vi "Joystick and Camera SHIH VPC- external Connection.vi"(0 "Motion in":refnum<class "Motion.lvclass">, 1 "XYZTheta":dbl[](array[numeric]), 2 "Measurement Point":string, 3 "Inital GO":bool=TRUE) -> (7 "Motion out":refnum<class "Motion.lvclass">, 8 "Sum":dbl[](array[numeric]), 9 "Gantry":dbl[](array[numeric]), 10 "error out":errorcluster)   [LabVIEW 2016]
uses:
  Classes/Controllers/Motion/Copy of Motion Folder/Motion.lvclass
  Classes/Controllers/Camera/Copy of Camera Folder/Machine Vision.ctl
  Classes/Controllers/Camera/Copy of Camera Folder/Camera.lvclass
  Classes/Controllers/Camera/Copy of Controller Folder/Controller.lvclass
panel:
  in  "case NN":dbl=0.001 format="%#_13g"
  in  "case NY":dbl=0.003 format="%#_13g"
  in  "?":bool
  in  "operation go":dbl[](array[numeric]) format="%#_9g"
  in  "case YN":dbl=0.01 format="%#_13g"
  in  "case YY":dbl=0.1 format="%#_13g"
  in  "?":bool=TRUE
  in  "step":dbl=15.0
  in  "Z go up":bool
  in  "Z go down":bool
  in  "Machine Vision":T1
  in  "object goes left":bool
  in  "object goes right":bool
  in  "object goes down":bool
  in  "object goes up":bool
  in  "Z go up 25 um":bool
  in  "Z go down 25 um":bool
  in  "Z go up 0.05 mm":bool
  in  "Z go down 0.05 mm":bool
  in  "Z go  up 0.1 mm":bool
  in  "Z go down 0.1 mm":bool
  in  "Machine Vision 2":T1=enum."None"
  out "Image 2":T2(plugin-control)
  out "Focus Index":dbl[](array[numeric])
  in  "interval":dbl=0.005
  out "Score":dbl[](array[numeric])
  out "Waveform Graph":dbl[](graph)
  in  "focus":bool
  out "Numeric":dbl
  in  "Go SUM":bool
  in  "Z Go":bool
  in  "Position":dbl
  in  "Go":bool
  in  "Joystick":bool
  in  "Stop":bool
  out "Image":T2(plugin-control)
  out "Camera":dbl[](array[numeric])
  # "mm"
  # "Y"
  # "Y"
  # "um"
  # "N"
  # "N"
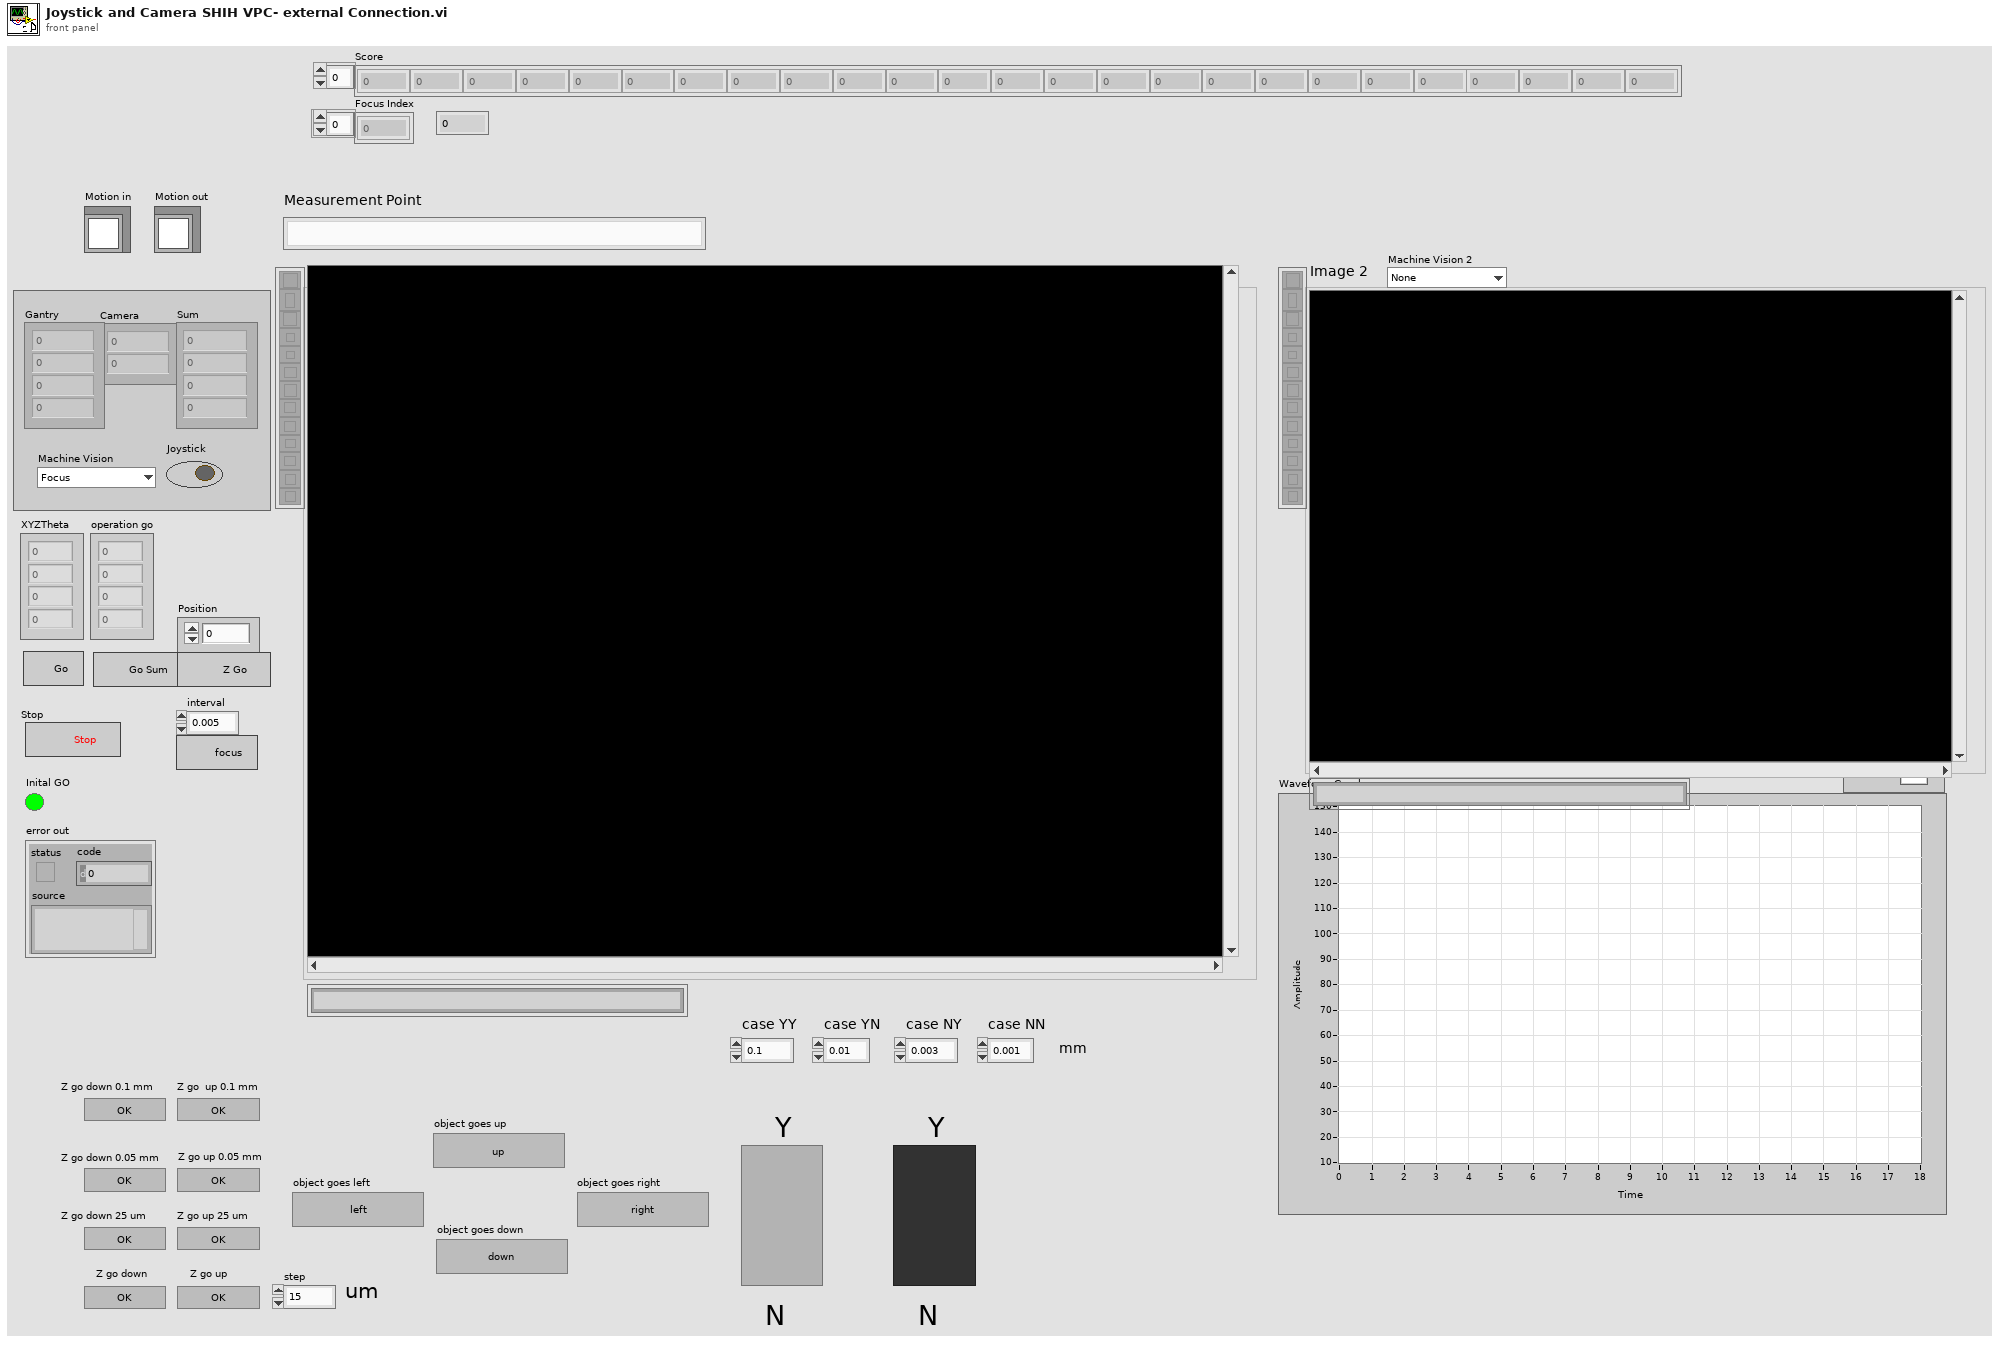
[diagram p1: front panel]
types:
  T1 = typedef "Camera.lvclass/Machine Vision.ctl" = enum16{"Focus", "chip cross", "LargeCircle", "None", "INTT HDI Mark", "INTT Sensor Cross", "INTT Chip Corner", "HPK Silicon", "circle"}
  T2 = typedef "IMAQ Image.ctl" = refnum<image>
  T3 = typedef "Controller.lvclass/Controllers.ctl" = cluster{"Copy of Motion.lvclass":refnum<class "Motion.lvclass">, "Copy of I-O.lvclass":refnum<class "I-O.lvclass">, "Copy of Dispenser.lvclass":refnum<class "Dispenser.lvclass">}
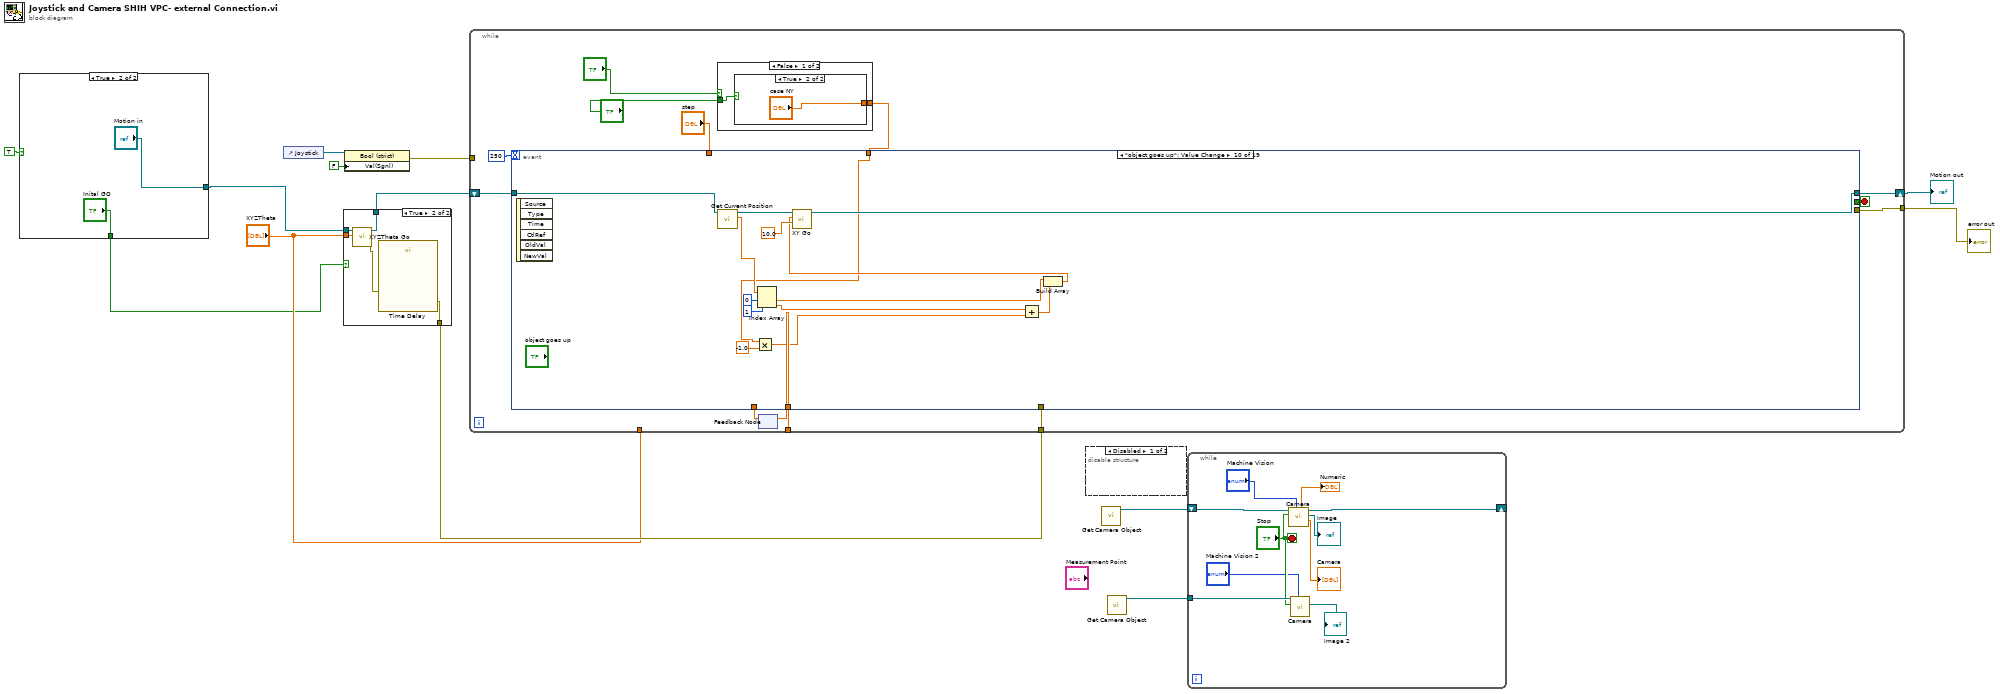
[diagram p0: block diagram]
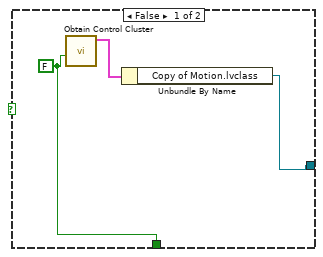
[diagram p3: hidden frame]
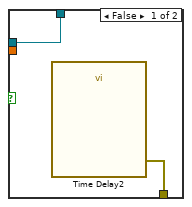
[diagram p4: hidden frame]
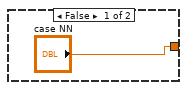
[diagram p5: hidden frame]
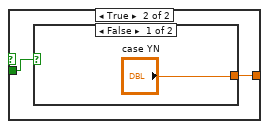
[diagram p6: hidden frame]
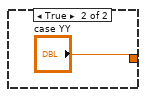
[diagram p7: hidden frame]
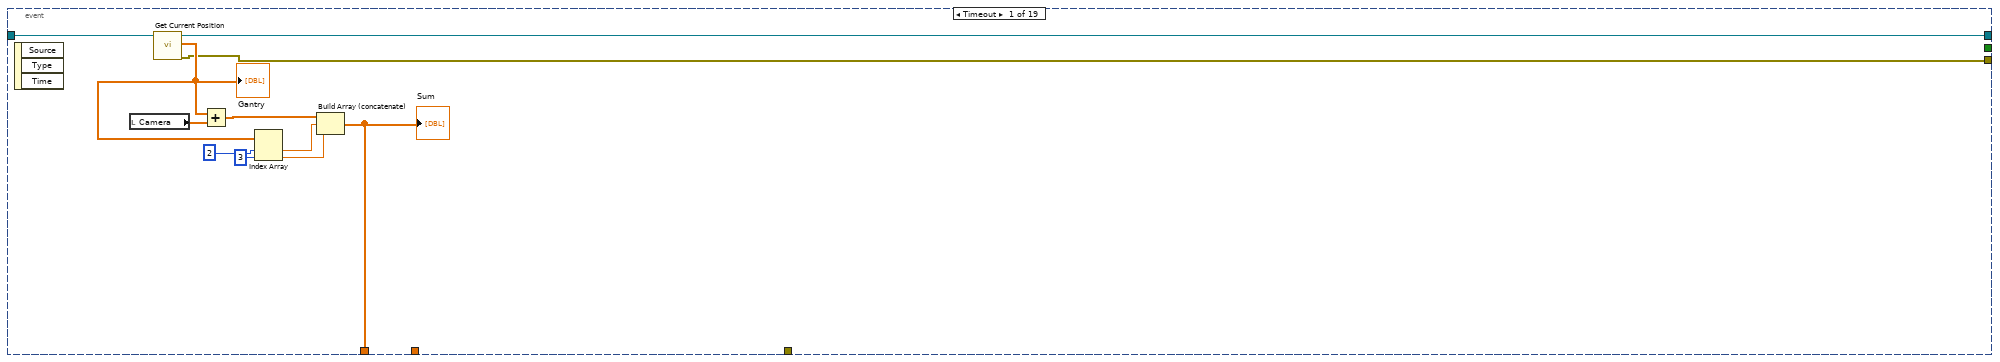
[diagram p8: hidden frame]
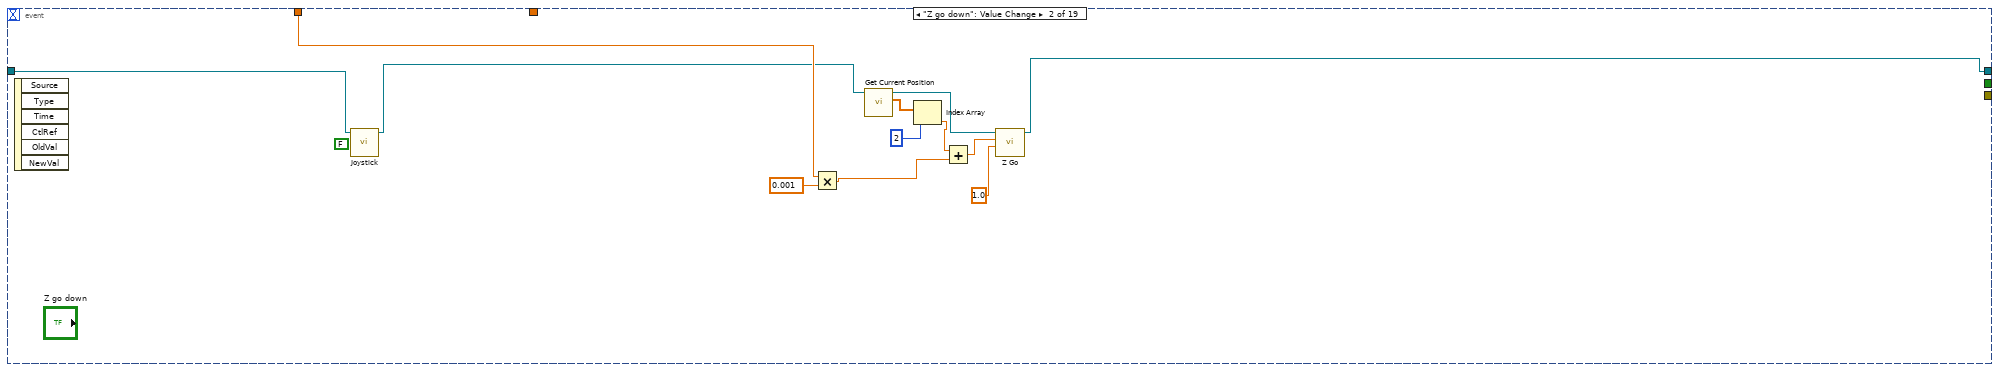
[diagram p9: hidden frame]
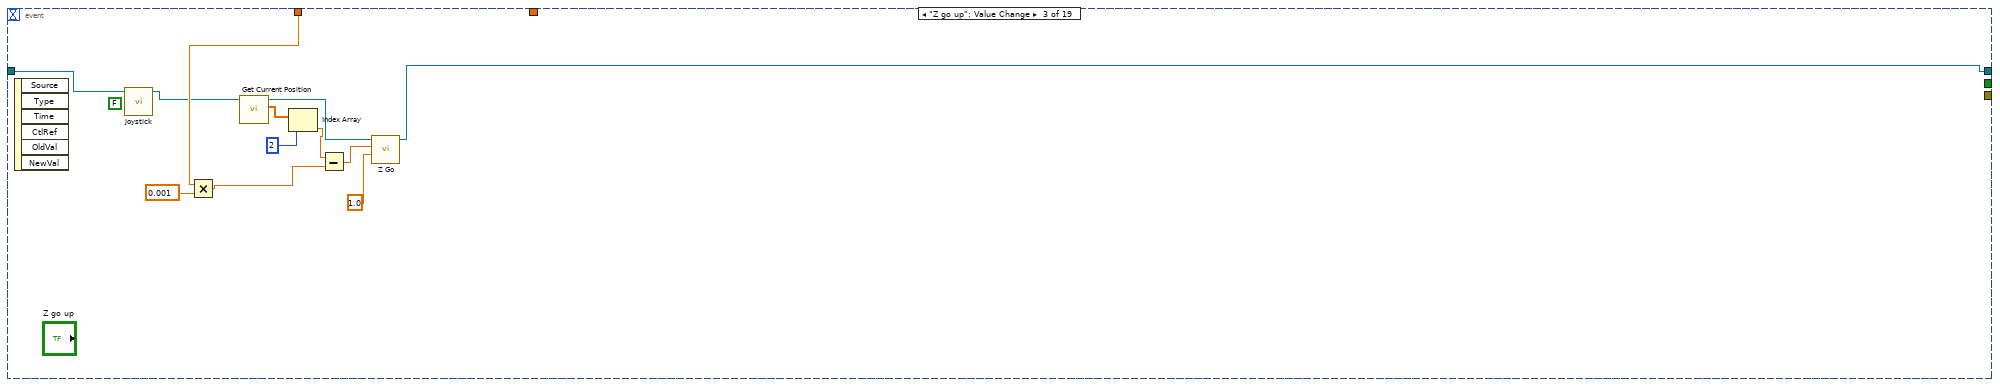
[diagram p10: hidden frame]
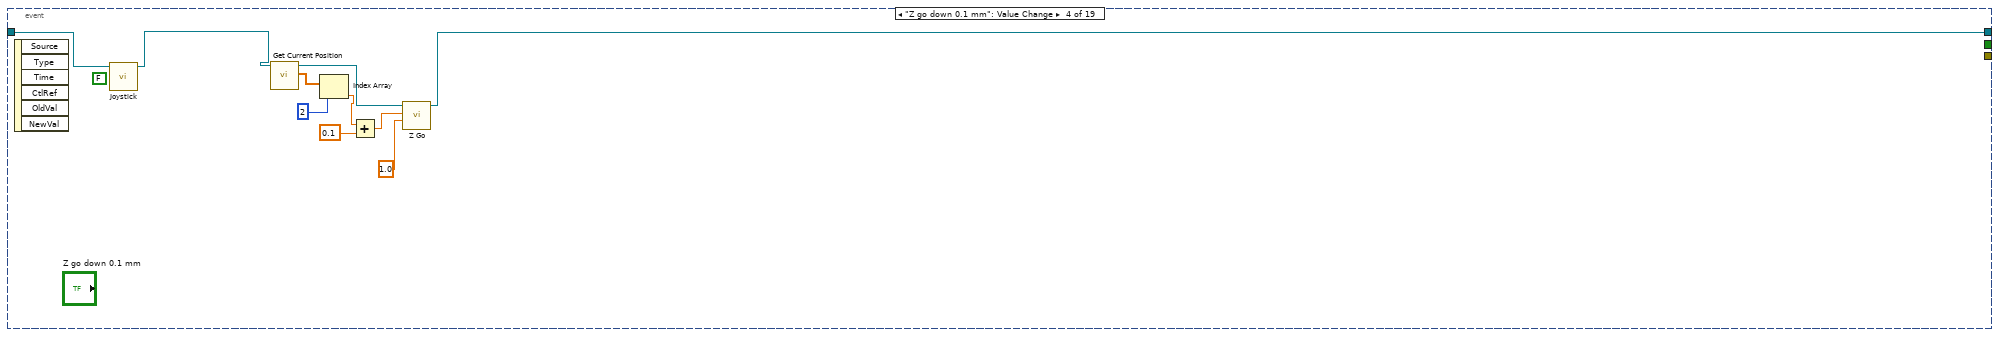
[diagram p11: hidden frame]
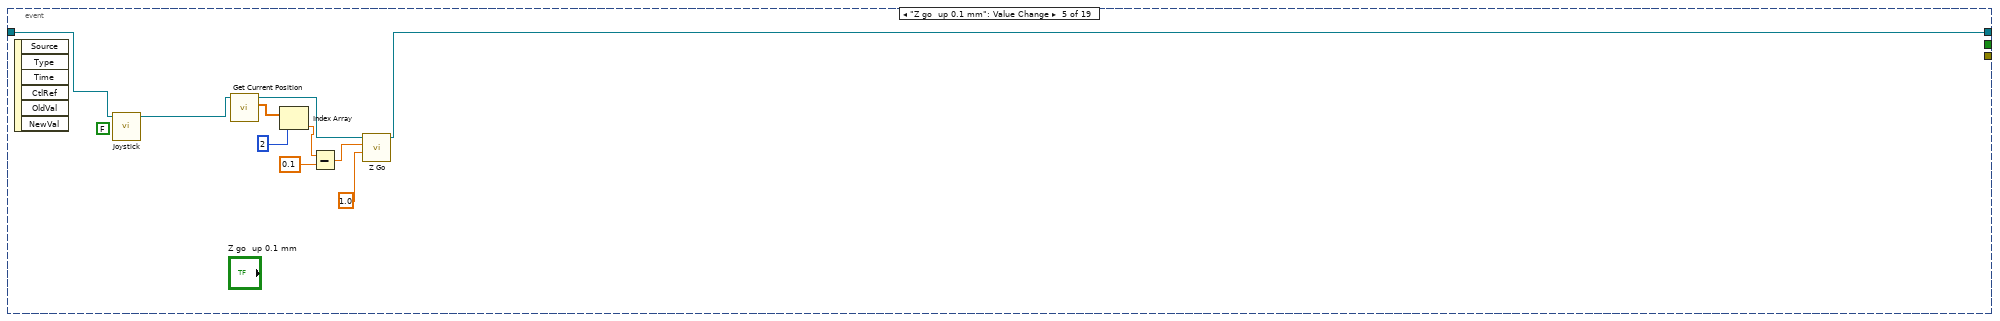
[diagram p12: hidden frame]
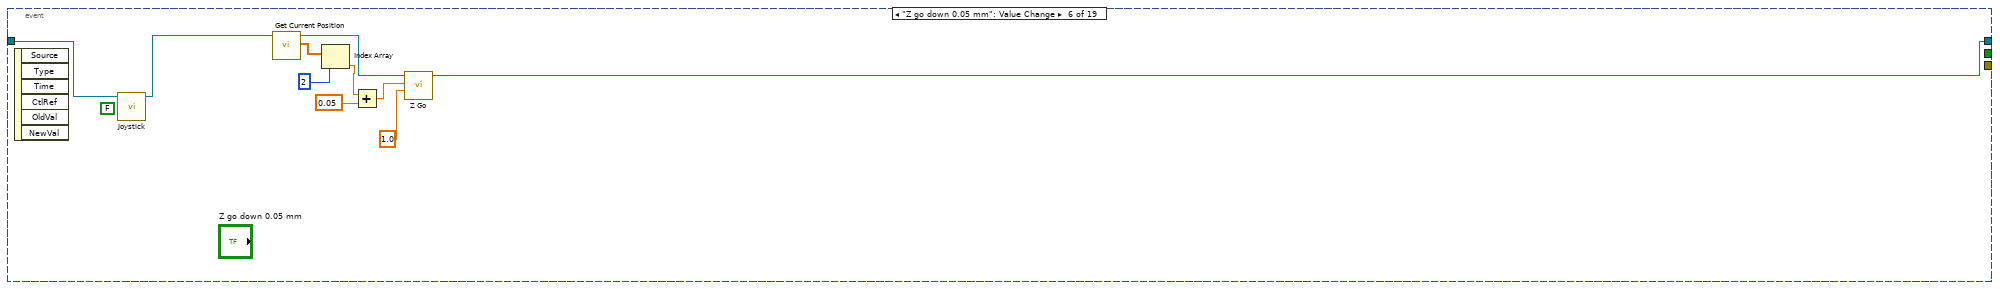
[diagram p13: hidden frame]
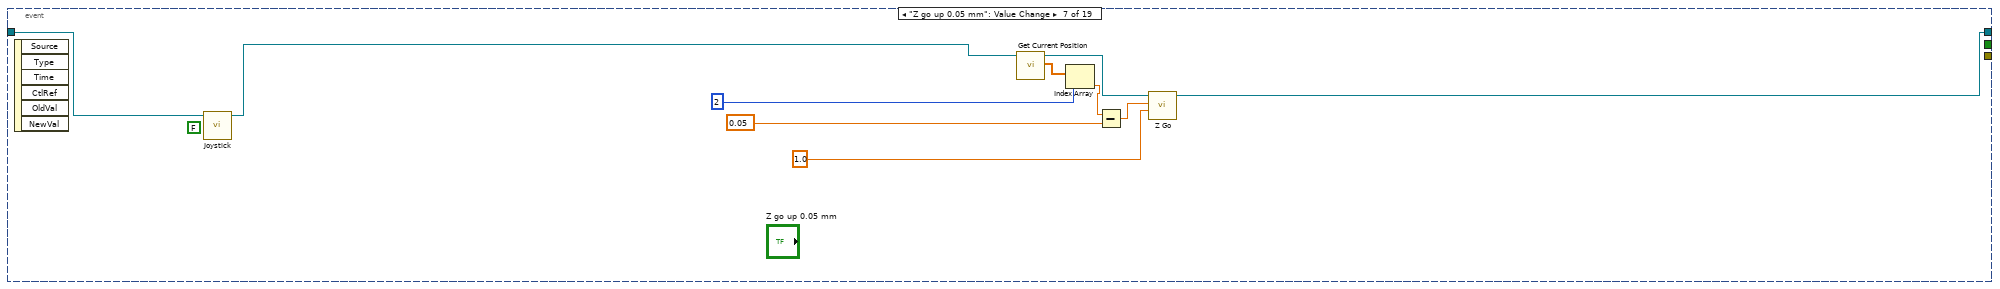
[diagram p14: hidden frame]
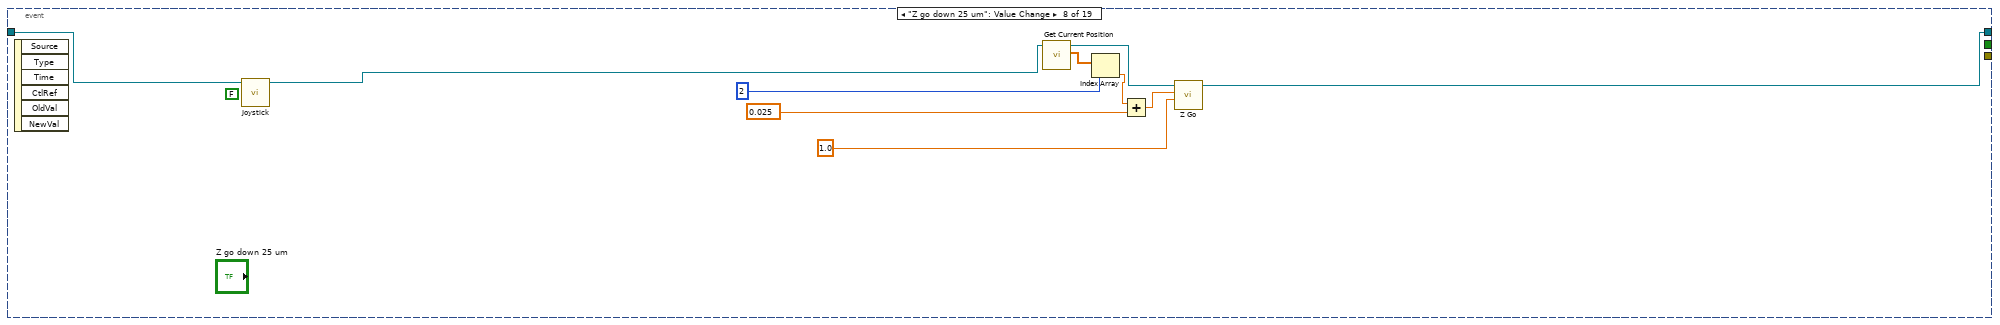
[diagram p15: hidden frame]
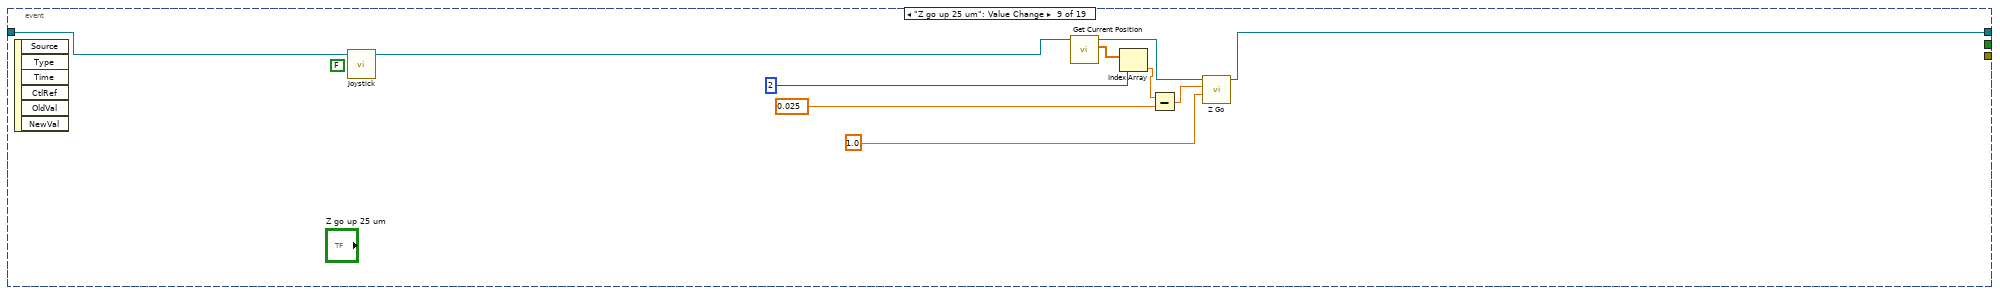
[diagram p16: hidden frame]
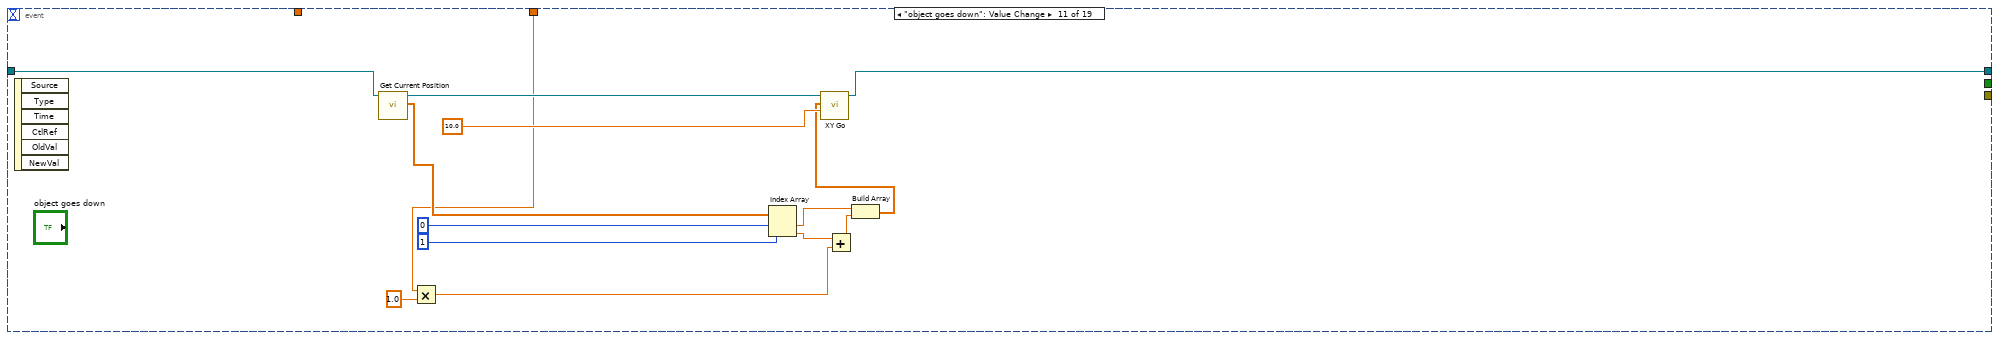
[diagram p17: hidden frame]
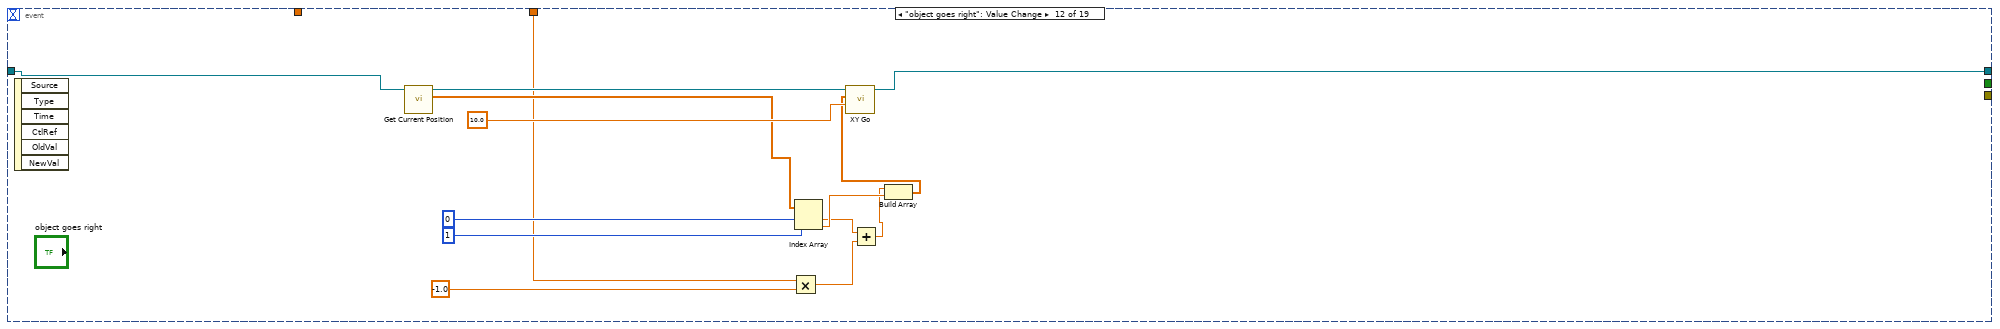
[diagram p18: hidden frame]
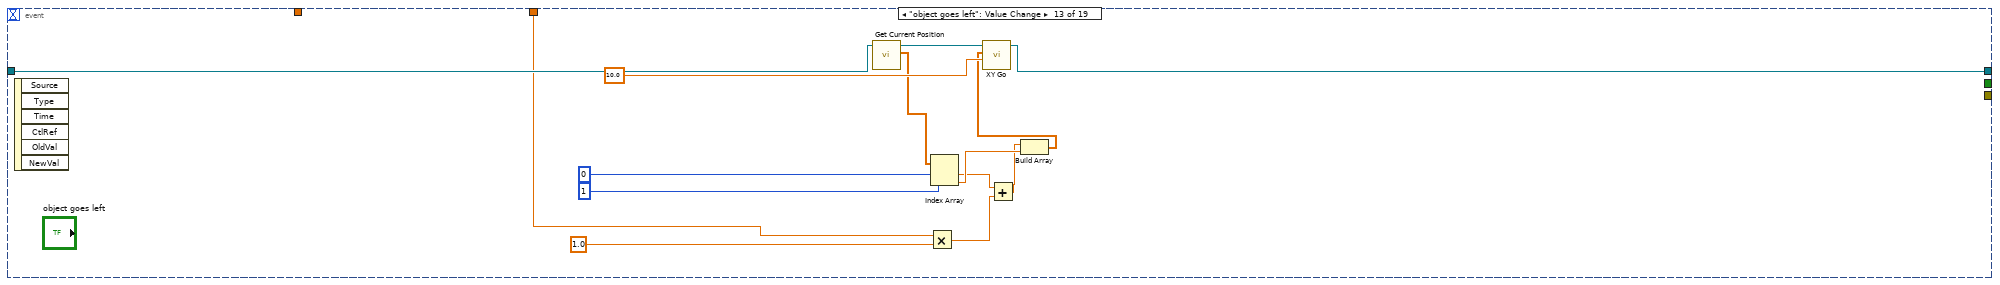
[diagram p19: hidden frame]
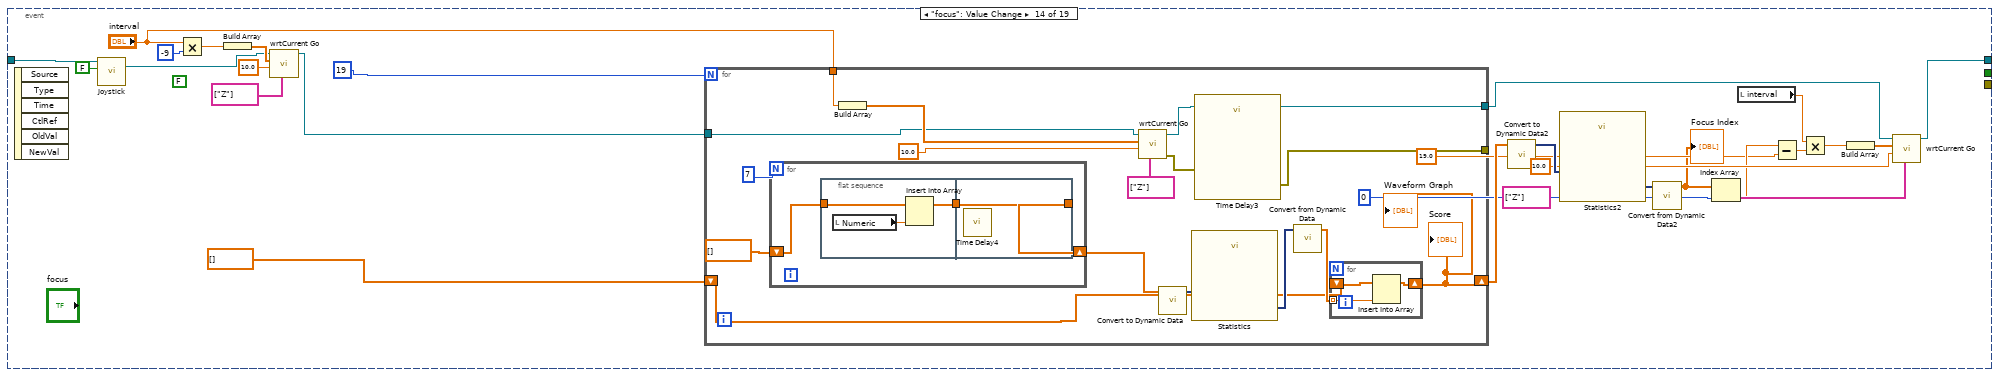
[diagram p20: hidden frame]
diagram:
  n1 = case shown="True" TRUE {
    tunnel: [w15 "Motion in"] -> w2
    tunnel: [w14 "Inital GO"] -> w1
    frame False {
      w14 = FALSE ("I/O")
      n2 = call "Obtain Control Cluster.vi"("I/O"=w14) -> ("Control Out"=w16:T3)  [unwired: 10 in]
      n3 = Unbundle By Name(w16) -> ("Copy of Motion.lvclass"=w15:refnum<class "Motion.lvclass">)
    }
    frame True {
    }
  }
  n4 = control-ref of="Joystick"() -> (w12:refnum<vi>)
  n5 = case shown="True" w1 {
    tunnel: w2 -> [w20 w25]
    tunnel: [w20 w24] -> w7
    tunnel: [w19 w22] -> w6
    tunnel: "XYZTheta" -> [_ w21]
    frame False {
      n6 = call "Time Delay2"() -> ("error out"=w19:errorcluster)  [unwired: 11 in]
    }
    frame True {
      n7 = call "XYZTheta Go.vi"("XYZTheta In"=w21, "Motion in"=w25) -> ("error out"=w23:errorcluster, "Motion out"=w24:refnum<class "Motion.lvclass">)  [unwired: 7 in, 1 out]
      n8 = call "Time Delay"("error in (no error)"=w23) -> ("error out"=w22:errorcluster)  [unwired: 10 in]
    }
  }
  n9 = property class="Bool (strict)"(reference=w12, "Val(Sgnl)"=FALSE ("Value (Signaling)")) -> (error out=w11:errorcluster)  [unwired: 1 in, 1 out]
  n10 = while {
    shift-right: [w34] -> w9
    shift-left: w7 -> [w35]
    tunnel: w11 -> [_]
    tunnel: [w33] -> w8
    tunnel: w6 -> [w32]
    tunnel: "XYZTheta" -> [_]
    tunnel: [w30] -> _
    stop <- w36 stop-if-true
    n11 = case shown="False" "?" {
      tunnel: [w38 w43] -> w27
      tunnel: "?" -> [w39 w42]
      frame False {
        n12 = case shown="True" w39 {
          tunnel: ["case NN" "case NY"] -> w38
          frame False {
          }
          frame True {
          }
        }
      }
      frame True {
        n13 = case shown="False" w42 {
          tunnel: ["case YN" "case YY"] -> w43
          frame False {
          }
          frame True {
          }
        }
      }
    }
    n14 = feedback #1() -> (w30:dbl[])  [unwired: 1 in]
    n15 = event shown="[9] \"object goes up\": Value Change" {
      selector: _ -> [_ _ _ _ _ _ _ _ _ _ _ _ _ _ _ _ _ _ _]
      dyn-events: _ -> [_ _ _ _ _ _ _ _ _ _ _ _ _ _ _ _ _ _ _]
      timeout: 250 -> [_ _ _ _ _ _ _ _ _ _ _ _ _ _ _ _ _ _ _]
      tunnel: [_ _ _ _ _ _ _ _ _ _ _ _ _ _ _ _ _ _ TRUE] -> w36
      tunnel: w35 -> [w55 w58 w70 w82 w92 w102 w112 w122 w132 w152 w162 w173 w187 w199 w254 w261 w285 w299 w309]
      tunnel: [w54 w59 w74 w83 w93 w103 w113 w123 w133 w151 w161 w174 w188 w198 w252 w260 w281 w305 w307] -> w34
      tunnel: [w49 _ _ _ _ _ _ _ _ _ _ _ _ _ w251 w258 w283 w300 _] -> w33
      tunnel: w32 -> [_ _ _ _ _ _ _ _ _ _ _ _ _ _ _ w257 w282 w301 _]
      tunnel: [w46 _ _ _ _ _ _ _ _ _ _ _ _ _ w250 w256 w280 w302 w306] -> w31
      tunnel: w30 -> [_ _ _ _ _ _ _ _ _ _ _ _ _ _ w250 w256 w280 w302 w306]
      tunnel: "step" -> [_ w60 w72 _ _ _ _ _ _ _ _ _ _ _ _ _ _ _ _]
      tunnel: w27 -> [_ _ _ _ _ _ _ _ _ w141 w155 w169 w183 _ _ _ _ _ _]
      event Timeout {
        n16 = event-data() -> ()  [unwired: 1 in, 3 out]
        n17 = local read "Camera"() -> (w56:dbl[])
        n18 = call-dynamic "Get Current Position.vi"("Motion in"=w55) -> ("error out"=w49:errorcluster, "XYZTheta Out"=w52:dbl[], "Motion out"=w54:refnum<class "Motion.lvclass">)  [unwired: 8 in]
        "Gantry" <- w52
        n19 = Add(x=w52, y=w56) -> (x+y=w53:dbl[])
        n20 = Index Array(array=w52, index #1=2 ("index"), index #2=3 ("index")) -> (element #1=w50:dbl, element #2=w47:dbl)
        n21 = Build Array (concatenate)(w53, w50, w47) -> (w46:dbl[])
        "Sum" <- w46
      }
      event "Z go down": Value Change {
        (unwired) FALSE ("Joystick")
        n22 = event-data() -> ()  [unwired: 1 in, 6 out]
        n23 = call-dynamic "Joystick.vi"("Motion in"=w58) -> ("Motion out"=w57:refnum<class "Motion.lvclass">)  [unwired: 9 in, 1 out]
        n24 = Multiply(x=w60, y=0.001) -> (x*y=w62:dbl)
        n25 = call-dynamic "Get Current Position.vi"("Motion in"=w57) -> ("XYZTheta Out"=w68:dbl[], "Motion out"=w66:refnum<class "Motion.lvclass">)  [unwired: 8 in, 1 out]
        n26 = Index Array(array=w68, index=2) -> (element=w63:dbl)
        n27 = Add(x=w63, y=w62) -> (x+y=w64:dbl)
        n28 = call-dynamic "Z Go.vi"("Speed"=1.0, "Position"=w64, "Motion in"=w66) -> ("Motion out"=w59:refnum<class "Motion.lvclass">)  [unwired: 7 in, 1 out]
      }
      event "Z go up": Value Change {
        (unwired) FALSE ("Joystick")
        n29 = event-data() -> ()  [unwired: 1 in, 6 out]
        n30 = call-dynamic "Joystick.vi"("Motion in"=w70) -> ("Motion out"=w69:refnum<class "Motion.lvclass">)  [unwired: 9 in, 1 out]
        n31 = Multiply(x=w72, y=0.001) -> (x*y=w73:dbl)
        n32 = call-dynamic "Get Current Position.vi"("Motion in"=w69) -> ("XYZTheta Out"=w80:dbl[], "Motion out"=w78:refnum<class "Motion.lvclass">)  [unwired: 8 in, 1 out]
        n33 = Index Array(array=w80, index=2) -> (element=w75:dbl)
        n34 = Subtract(x=w75, y=w73) -> (x-y=w76:dbl)
        n35 = call-dynamic "Z Go.vi"("Speed"=1.0, "Position"=w76, "Motion in"=w78) -> ("Motion out"=w74:refnum<class "Motion.lvclass">)  [unwired: 7 in, 1 out]
      }
      event "Z go down 0.1 mm": Value Change {
        (unwired) FALSE ("Joystick")
        n36 = event-data() -> ()  [unwired: 1 in, 6 out]
        n37 = call-dynamic "Joystick.vi"("Motion in"=w82) -> ("Motion out"=w81:refnum<class "Motion.lvclass">)  [unwired: 9 in, 1 out]
        n38 = call-dynamic "Get Current Position.vi"("Motion in"=w81) -> ("XYZTheta Out"=w90:dbl[], "Motion out"=w88:refnum<class "Motion.lvclass">)  [unwired: 8 in, 1 out]
        n39 = Index Array(array=w90, index=2) -> (element=w85:dbl)
        n40 = Add(x=w85, y=0.1) -> (x+y=w86:dbl)
        n41 = call-dynamic "Z Go.vi"("Speed"=1.0, "Position"=w86, "Motion in"=w88) -> ("Motion out"=w83:refnum<class "Motion.lvclass">)  [unwired: 7 in, 1 out]
      }
      event "Z go  up 0.1 mm": Value Change {
        (unwired) FALSE ("Joystick")
        n42 = event-data() -> ()  [unwired: 1 in, 6 out]
        n43 = call-dynamic "Joystick.vi"("Motion in"=w92) -> ("Motion out"=w91:refnum<class "Motion.lvclass">)  [unwired: 9 in, 1 out]
        n44 = call-dynamic "Get Current Position.vi"("Motion in"=w91) -> ("XYZTheta Out"=w100:dbl[], "Motion out"=w98:refnum<class "Motion.lvclass">)  [unwired: 8 in, 1 out]
        n45 = Index Array(array=w100, index=2) -> (element=w95:dbl)
        n46 = Subtract(x=w95, y=0.1) -> (x-y=w96:dbl)
        n47 = call-dynamic "Z Go.vi"("Speed"=1.0, "Position"=w96, "Motion in"=w98) -> ("Motion out"=w93:refnum<class "Motion.lvclass">)  [unwired: 7 in, 1 out]
      }
      event "Z go down 0.05 mm": Value Change {
        (unwired) FALSE ("Joystick")
        n48 = event-data() -> ()  [unwired: 1 in, 6 out]
        n49 = call-dynamic "Joystick.vi"("Motion in"=w102) -> ("Motion out"=w101:refnum<class "Motion.lvclass">)  [unwired: 9 in, 1 out]
        n50 = call-dynamic "Get Current Position.vi"("Motion in"=w101) -> ("XYZTheta Out"=w110:dbl[], "Motion out"=w108:refnum<class "Motion.lvclass">)  [unwired: 8 in, 1 out]
        n51 = Index Array(array=w110, index=2) -> (element=w105:dbl)
        n52 = Add(x=w105, y=0.05) -> (x+y=w106:dbl)
        n53 = call-dynamic "Z Go.vi"("Speed"=1.0, "Position"=w106, "Motion in"=w108) -> ("Motion out"=w103:refnum<class "Motion.lvclass">)  [unwired: 7 in, 1 out]
      }
      event "Z go up 0.05 mm": Value Change {
        (unwired) FALSE ("Joystick")
        n54 = event-data() -> ()  [unwired: 1 in, 6 out]
        n55 = call-dynamic "Joystick.vi"("Motion in"=w112) -> ("Motion out"=w111:refnum<class "Motion.lvclass">)  [unwired: 9 in, 1 out]
        n56 = call-dynamic "Get Current Position.vi"("Motion in"=w111) -> ("XYZTheta Out"=w120:dbl[], "Motion out"=w118:refnum<class "Motion.lvclass">)  [unwired: 8 in, 1 out]
        n57 = Index Array(array=w120, index=2) -> (element=w115:dbl)
        n58 = Subtract(x=w115, y=0.05) -> (x-y=w116:dbl)
        n59 = call-dynamic "Z Go.vi"("Speed"=1.0, "Position"=w116, "Motion in"=w118) -> ("Motion out"=w113:refnum<class "Motion.lvclass">)  [unwired: 7 in, 1 out]
      }
      event "Z go down 25 um": Value Change {
        (unwired) FALSE ("Joystick")
        n60 = event-data() -> ()  [unwired: 1 in, 6 out]
        n61 = call-dynamic "Joystick.vi"("Motion in"=w122) -> ("Motion out"=w121:refnum<class "Motion.lvclass">)  [unwired: 9 in, 1 out]
        n62 = call-dynamic "Get Current Position.vi"("Motion in"=w121) -> ("XYZTheta Out"=w130:dbl[], "Motion out"=w128:refnum<class "Motion.lvclass">)  [unwired: 8 in, 1 out]
        n63 = Index Array(array=w130, index=2) -> (element=w125:dbl)
        n64 = Add(x=w125, y=0.025) -> (x+y=w126:dbl)
        n65 = call-dynamic "Z Go.vi"("Speed"=1.0, "Position"=w126, "Motion in"=w128) -> ("Motion out"=w123:refnum<class "Motion.lvclass">)  [unwired: 7 in, 1 out]
      }
      event "Z go up 25 um": Value Change {
        (unwired) FALSE ("Joystick")
        n66 = event-data() -> ()  [unwired: 1 in, 6 out]
        n67 = call-dynamic "Joystick.vi"("Motion in"=w132) -> ("Motion out"=w131:refnum<class "Motion.lvclass">)  [unwired: 9 in, 1 out]
        n68 = call-dynamic "Get Current Position.vi"("Motion in"=w131) -> ("XYZTheta Out"=w140:dbl[], "Motion out"=w138:refnum<class "Motion.lvclass">)  [unwired: 8 in, 1 out]
        n69 = Index Array(array=w140, index=2) -> (element=w135:dbl)
        n70 = Subtract(x=w135, y=0.025) -> (x-y=w136:dbl)
        n71 = call-dynamic "Z Go.vi"("Speed"=1.0, "Position"=w136, "Motion in"=w138) -> ("Motion out"=w133:refnum<class "Motion.lvclass">)  [unwired: 7 in, 1 out]
      }
      event "object goes up": Value Change {
        n72 = event-data() -> ()  [unwired: 1 in, 6 out]
        n73 = call-dynamic "Get Current Position.vi"("Motion in"=w152) -> ("XYZTheta Out"=w150:dbl[], "Motion out"=w154:refnum<class "Motion.lvclass">)  [unwired: 8 in, 1 out]
        n74 = Multiply(x=w141, y=-1.0) -> (x*y=w146:dbl)
        n75 = Index Array(array=w150, index #1=0 ("index"), index #2=1 ("index")) -> (element #1=w144:dbl, element #2=w143:dbl)
        n76 = Add(x=w143, y=w146) -> (x+y=w142:dbl)
        n77 = Build Array(w144, w142) -> (w147:dbl[])
        n78 = call-dynamic "XY Go.vi"("Speed"=10.0, "XY"=w147, "Motion in"=w154) -> ("Motion out"=w151:refnum<class "Motion.lvclass">)  [unwired: 7 in, 1 out]
      }
      event "object goes down": Value Change {
        n79 = event-data() -> ()  [unwired: 1 in, 6 out]
        n80 = call-dynamic "Get Current Position.vi"("Motion in"=w162) -> ("XYZTheta Out"=w166:dbl[], "Motion out"=w168:refnum<class "Motion.lvclass">)  [unwired: 8 in, 1 out]
        n81 = Multiply(x=w155, y=1.0) -> (x*y=w160:dbl)
        n82 = Index Array(array=w166, index #1=0 ("index"), index #2=1 ("index")) -> (element #1=w158:dbl, element #2=w157:dbl)
        n83 = Add(x=w157, y=w160) -> (x+y=w156:dbl)
        n84 = Build Array(w158, w156) -> (w163:dbl[])
        n85 = call-dynamic "XY Go.vi"("Speed"=10.0, "XY"=w163, "Motion in"=w168) -> ("Motion out"=w161:refnum<class "Motion.lvclass">)  [unwired: 7 in, 1 out]
      }
      event "object goes right": Value Change {
        n86 = event-data() -> ()  [unwired: 1 in, 6 out]
        n87 = call-dynamic "Get Current Position.vi"("Motion in"=w173) -> ("XYZTheta Out"=w180:dbl[], "Motion out"=w182:refnum<class "Motion.lvclass">)  [unwired: 8 in, 1 out]
        n88 = Multiply(x=w169, y=-1.0) -> (x*y=w176:dbl)
        n89 = Index Array(array=w180, index #1=0 ("index"), index #2=1 ("index")) -> (element #1=w171:dbl, element #2=w172:dbl)
        n90 = Add(x=w171, y=w176) -> (x+y=w170:dbl)
        n91 = Build Array(w170, w172) -> (w177:dbl[])
        n92 = call-dynamic "XY Go.vi"("Speed"=10.0, "XY"=w177, "Motion in"=w182) -> ("Motion out"=w174:refnum<class "Motion.lvclass">)  [unwired: 7 in, 1 out]
      }
      event "object goes left": Value Change {
        n93 = event-data() -> ()  [unwired: 1 in, 6 out]
        n94 = call-dynamic "Get Current Position.vi"("Motion in"=w187) -> ("XYZTheta Out"=w194:dbl[], "Motion out"=w196:refnum<class "Motion.lvclass">)  [unwired: 8 in, 1 out]
        n95 = Multiply(x=w183, y=1.0) -> (x*y=w190:dbl)
        n96 = Index Array(array=w194, index #1=0 ("index"), index #2=1 ("index")) -> (element #1=w185:dbl, element #2=w186:dbl)
        n97 = Add(x=w185, y=w190) -> (x+y=w184:dbl)
        n98 = Build Array(w184, w186) -> (w191:dbl[])
        n99 = call-dynamic "XY Go.vi"("Speed"=10.0, "XY"=w191, "Motion in"=w196) -> ("Motion out"=w188:refnum<class "Motion.lvclass">)  [unwired: 7 in, 1 out]
      }
      event "focus": Value Change {
        (unwired) FALSE ("Joystick")
        n100 = event-data() -> ()  [unwired: 1 in, 6 out]
        n101 = call-dynamic "Joystick.vi"("Joystick"=FALSE, "Motion in"=w199) -> ("Motion out"=w201:refnum<class "Motion.lvclass">)  [unwired: 8 in, 1 out]
        n102 = Multiply(x="interval", y=-9) -> (x*y=w216:dbl)
        n103 = Build Array(w216) -> (w218:dbl[])
        n104 = call-dynamic "wrtCurrent Go.vi"("axis names"=string[] ["Z"] ("Axis"), "Speed"=10.0, "distances"=w218, "Motion in"=w201) -> ("Motion out"=w222:refnum<class "Motion.lvclass">)  [unwired: 6 in, 1 out]
        n105 = for {
          N: 19 -> [_]
          tunnel: w222 -> [w224]
          tunnel: [w228] -> w208
          shift-right: [w225] -> w214
          shift-left: dbl[] [] -> [w226]
          tunnel: "interval" -> [w231]
          tunnel: [w227] -> _
          n106 = for {
            N: 7 -> [_]
            shift-right: [w245] -> w236
            shift-left: dbl[] [] -> [w244]
            n107 = flat-sequence {
              tunnel: w244 -> [w247]
              tunnel: [w248] -> w243
              tunnel: [w249] -> w245
              tunnel: w243 -> [w249]
              frame #0 {
                n108 = local read "Numeric"() -> (w246:dbl)
                n109 = Insert Into Array(array=w247, new element=w246) -> (w248:dbl[])  [unwired: 1 in]
              }
              frame #1 {
                n110 = call "Time Delay4"() -> ()  [unwired: 11 in, 1 out]
              }
            }
          }
          n111 = Build Array(w231) -> (w230:dbl[])
          n112 = call-dynamic "wrtCurrent Go.vi"("axis names"=string[] ["Z"] ("Axis"), "Speed"=10.0, "distances"=w230, "Motion in"=w224) -> ("error out"=w237:errorcluster, "Motion out"=w228:refnum<class "Motion.lvclass">)  [unwired: 6 in]
          n113 = call "Convert to Dynamic Data"("Array"=w236) -> ("Dynamic Data Type"=w235:dynamicdata)  [unwired: 3 in]
          n114 = call "Statistics"("Signals"=w235) -> ("Arithmetic Mean"=w233:dynamicdata)  [unwired: 25 in, 1 out]
          n115 = call "Time Delay3"("error in (no error)"=w237) -> ("error out"=w227:errorcluster)  [unwired: 10 in]
          n116 = call "Convert from Dynamic Data"("Dynamic Data Type"=w233) -> ("Array"=w229:dbl[])  [unwired: 3 in]
          n117 = for {
            tunnel: w229 -> [w242] mode=indexing
            shift-right: [w241] -> w225
            shift-left: w226 -> [w240]
            n118 = Insert Into Array(array=w240, new element=w242) -> (w241:dbl[])  [unwired: 1 in]
          }
          "Score" <- w225
          "Waveform Graph" <- w225
        }
        n119 = call "Convert to Dynamic Data2"("Array"=w214) -> ("Dynamic Data Type"=w213:dynamicdata)  [unwired: 3 in]
        n120 = call "Statistics2"("Signals"=w213) -> ("Index of Max"=w212:dynamicdata)  [unwired: 25 in, 1 out]
        n121 = call "Convert from Dynamic Data2"("Dynamic Data Type"=w212) -> ("Array"=w200:dbl[])  [unwired: 3 in]
        "Focus Index" <- w200
        n122 = Index Array(array=w200, index=0) -> (element=w203:dbl)
        n123 = local read "interval"() -> (w206:dbl)
        n124 = Subtract(x=w203, y=19.0 ("x")) -> (x-y=w207:dbl)
        n125 = Multiply(x=w206, y=w207) -> (x*y=w205:dbl)
        n126 = Build Array(w205) -> (w204:dbl[])
        n127 = call-dynamic "wrtCurrent Go.vi"("axis names"=string[] ["Z"] ("Axis"), "Speed"=10.0, "distances"=w204, "Motion in"=w208) -> ("Motion out"=w198:refnum<class "Motion.lvclass">)  [unwired: 6 in, 1 out]
      }
      event "Joystick": Value Change {
        n128 = event-data() -> ()  [unwired: 1 in, 6 out]
        n129 = call-dynamic "Joystick.vi"("Joystick"="Joystick", "Motion in"=w254) -> ("error out"=w251:errorcluster, "Motion out"=w252:refnum<class "Motion.lvclass">)  [unwired: 8 in]
      }
      event "Go": Value Change {
        n130 = event-data() -> ()  [unwired: 1 in, 6 out]
        n131 = flat-sequence {
          tunnel: w261 -> [w263]
          tunnel: [w262] -> w259
          tunnel: [w268] -> w260
          tunnel: w259 -> [w271]
          tunnel: [w267] -> w258
          tunnel: w257 -> [w266]
          tunnel: "operation go" -> [w265]
          frame #0 {
            n132 = call-dynamic "Joystick.vi"("Joystick"=FALSE, "Motion in"=w263) -> ("Motion out"=w262:refnum<class "Motion.lvclass">)  [unwired: 8 in, 1 out]
          }
          frame #1 {
            n133 = for {
              tunnel: w265 -> [w277] mode=indexing
              tunnel: [w275] -> w270 mode=indexing
              shift-right: [w273] -> w269
              shift-left: w271 -> [w274]
              i -> [w279]
              n134 = Equal To 0?(x=w277) -> (x = 0?=w278:bool)
              n135 = call-dynamic "Get Current Position.vi"("Motion in"=w274) -> ("XYZTheta Out"=w272:dbl[], "Motion out"=w273:refnum<class "Motion.lvclass">)  [unwired: 8 in, 1 out]
              n136 = Index Array(array=w272, index=w279) -> (element=w276:dbl)
              n137 = Select(t=w276, s=w278, f=w277) -> (s? t:f=w275:dbl)
            }
            n138 = call "XYZTheta Go.vi"("error in (no error)"=w266, "XYZTheta In"=w270, "Motion in"=w269) -> ("error out"=w267:errorcluster, "Motion out"=w268:refnum<class "Motion.lvclass">)  [unwired: 6 in, 1 out]
          }
        }
      }
      event "Go SUM": Value Change {
        n139 = event-data() -> ()  [unwired: 1 in, 6 out]
        n140 = flat-sequence {
          tunnel: w285 -> [w287]
          tunnel: [w286] -> w284
          tunnel: w284 -> [w293]
          tunnel: [w291] -> w283
          tunnel: w282 -> [w292]
          tunnel: w280 -> [w296]
          tunnel: [w290] -> w281
          frame #0 {
            n141 = call-dynamic "Joystick.vi"("Joystick"=FALSE, "Motion in"=w287) -> ("Motion out"=w286:refnum<class "Motion.lvclass">)  [unwired: 8 in, 1 out]
          }
          frame #1 {
            n142 = Array Subset(array=w296, index=0, length=2) -> (w289:dbl[])
            n143 = call-dynamic "XY Go.vi"("error in (no error)"=w292, "Speed"=10.0, "XY"=w289, "Motion in"=w293) -> ("error out"=w291:errorcluster, "Motion out"=w290:refnum<class "Motion.lvclass">)  [unwired: 6 in]
          }
        }
      }
      event "Z Go": Value Change {
        (unwired) FALSE ("Joystick")
        n144 = event-data() -> ()  [unwired: 1 in, 6 out]
        n145 = call-dynamic "Joystick.vi"("Motion in"=w299) -> ("Motion out"=w298:refnum<class "Motion.lvclass">)  [unwired: 9 in, 1 out]
        n146 = call-dynamic "Z Go.vi"("error in (no error)"=w301, "Speed"=2.0, "Position"="Position", "Motion in"=w298) -> ("error out"=w300:errorcluster, "Motion out"=w305:refnum<class "Motion.lvclass">)  [unwired: 6 in]
      }
      event "Stop": Value Change {
        n147 = event-data() -> ()  [unwired: 1 in, 5 out]
        n148 = call-dynamic "Joystick.vi"("Joystick"=FALSE, "Motion in"=w309) -> ("Motion out"=w307:refnum<class "Motion.lvclass">)  [unwired: 8 in, 1 out]
      }
    }
    n149 = feedback-in #1(w31) -> ()
  }
  "error out" <- w8
  "Motion out" <- w9
  n150 = disable-structure shown="Disabled" {
    frame Disabled {
    }
    frame Enabled {
    }
  }
  n151 = call "Get Camera Object.vi"() -> ("Camera out"=w10:refnum<class "Camera.lvclass">)  [unwired: 10 in, 1 out]
  n152 = call "Get Camera Object.vi"() -> ("Camera out"=w4:refnum<class "Camera.lvclass">)  [unwired: 10 in, 1 out]
  n153 = while {
    shift-right: [w319] -> _
    shift-left: w10 -> [w320]
    tunnel: w4 -> [w315]
    stop <- "Stop" stop-if-true
    n154 = call "Camera.vi"("Machine Vision"="Machine Vision", "Stop"="Stop", "Camera in"=w320) -> ("Camera"=→"Camera":dbl[], "Image"=→"Image":T2, "Camera out"=w319:refnum<class "Camera.lvclass">, "Numeric"=→"Numeric":dbl)  [unwired: 2 in, 3 out]
    n155 = call "Camera.vi"("Machine Vision"="Machine Vision 2", "Stop"="Stop", "Camera in"=w315) -> ("Image"=→"Image 2":T2)  [unwired: 2 in, 6 out]
  }
